vi "IR Opo Main.vi"() -> ()   [LabVIEW 2016]
uses:
  System.Windows.Forms
  D:/Fabrizio/Labview Projects/IR OPO Controller/Branches/XPS version/uc480DotNet.dll
  uc480DotNet.dll
  <vilib>/Utility/miscctls.llb/LVBoundsTypeDef.ctl
  <vilib>/Utility/config.llb/Write Key (Double).vi
  <vilib>/Utility/config.llb/Write Key (I32).vi
  <vilib>/Utility/config.llb/Read Key (String).vi
  <vilib>/Utility/config.llb/Read Key (Double).vi
  <vilib>/Utility/config.llb/Read Key (I32).vi
  <vilib>/vision/NI_Vision_Development_Module.lvlib
  <vilib>/Utility/config.llb/NI_LVConfig.lvlib
  OPOTEK.dll
panel:
  in  "Acceleration \n(mm/s²)":dbl=20.0
  out "Camera Status":string="Load parameter"
  in  "Save configuration":bool
  in  "Stages status":bool
  in  "Transparency":u8 max=80 step=1
  in  "Overlay MSI Image":bool
  in  "Home Axes":bool
  in  "Tune":bool
  out "Axis 2 Offset":dbl
  out "Axis 1 Offset":dbl
  out "Acceleration":dbl
  out "Velocity":dbl
  in  "Axis Initial Parameters":T1={"Velocity (units/seconds)"=1.0, "Acceleration (units/seconds²)"=20.0, "Minimum Jerk Time (seconds)"=0.005, "Maximum Jerk Time (seconds)"=0.009} {"Maximum Jerk Time (seconds)" format="%.6e"; "Minimum Jerk Time (seconds)" format="%.6e"; "Acceleration (units/seconds²)" format="%.6e"; "Velocity (units/seconds)" format="%.6e"}
  out "Axis 2":string
  out "Axis 1":string
  out "XPS_Address":string
  in  "Axes Manual Control":bool
  out "ROI Area \n(mm2)":dbl=4.035870075999999
  out "Default Wavelenght":i32
  out "Laser on/off array":bool[][](array[boolean])
  out "Commands array":string[][](array[string])
  in  "Exit Camera":bool
  in  "Width (µm)":i32=240
  in  "Y offset":i32=406 step=1
  in  "X offset":i32=693 step=1
  out "Processi time (sec)":i32=117
  in  "Processing time unit":string(combo)="sec"
  out "Process time":dbl=117.0
  in  "Mode":i32(ring) items=["RGB 32"=0, "RGB 24"=1, "Y8 Monochrom"=6]
  in  "Camera":refnum<k24>(container)
  in  "Init Camera":bool
  in  "Start Live":bool
  in  "Stop Live":bool
  in  "Load Parameter":bool
  out "Error Out":errorcluster caption="error"
  out "Bits/Pixel":i32=32
  out "Width":i32=1280
  out "Height":i32=1024
  out "Serial Number":string="4102944807"
  in  "Camera ID":i32
  in  "Zoom":dbl(ring)=1.5 items=["4X"=4.0, "2X"=2.0, "1.5X"=1.5, "1.25X"=1.25, "1X"=1.0]
  in  "Gain Boost":bool=TRUE
  in  "Snapshot":bool
  out "Output":picture
  in  "Exposure":dbl(slide)=99.80425000000001 min=0.049933333333333337 max=99.9166 step=0.049933333333333337 scale=0.049933333333333337..99.9166 scale format="%#.3g"
  in  "Framerate":dbl(slide)=10.002522802986672 min=0.5926462556135453 max=18.75159388548027 step=0.01754124778810128 scale=0.5926462556135453..18.75159388548027 scale format="%#.3g"
  in  "Pixelclock":i32(slide)=24 min=5 max=40 step=1 scale=5.0..40.0
  in  "error in (no error)":errorcluster
  out "error out":errorcluster
  in  "Precision (%)":dbl=1.0 min=1.0 max=100.0 step=1.0 format="%#_3g"
  out "Time array":dbl[][](array[numeric])
  in  "Process Image":bool
  in  "Pixel size":dbl=12.19 step=0.01
  in  "Speed (µm/s)":i32=1000
  in  "Heigth (µm)":i32=240
  in  "Height  step \ndivider":i32=2
  out "ROI container\nheigth (µm)":i32=2267
  out "ROI container\nwidth (µm)":i32=2267
  out "Source":T2(plugin-control)
  in  "Open \nManual":bool
  in  "Capture":bool
  out "Log":string
  out "Laser Operation":bool
  in  "Alignment \ndiode":bool
  in  "LASER":bool
  in  "LAMP":bool
  in  "Wavelength":dbl=2940.0 min=2600.0 max=3200.0 step=1.0
  out "error_Code 3":i32
  in  "Repetition \nRate":enum16{"1", "2", "5", "10", "20"}(ring)=enum."20"
  in  "Flash lamp - Q Switch delay (%)":i16(slide) min=0 max=100 scale=0.0..100.0 scale format="%#.1f"
  out "error_Code 2":i32
  out "Max":dbl=3200.0
  out "Min":dbl=2600.0
  out "error_Code":i32
  out "laserCOMPort":i32
  out "motorCOMPort":i32
  in  "EXIT":bool
  # "Laser Control"
  # "Stages Control"
  # "Camera Control"
  # "ROI Processing"
  # "Laser spot size and position"
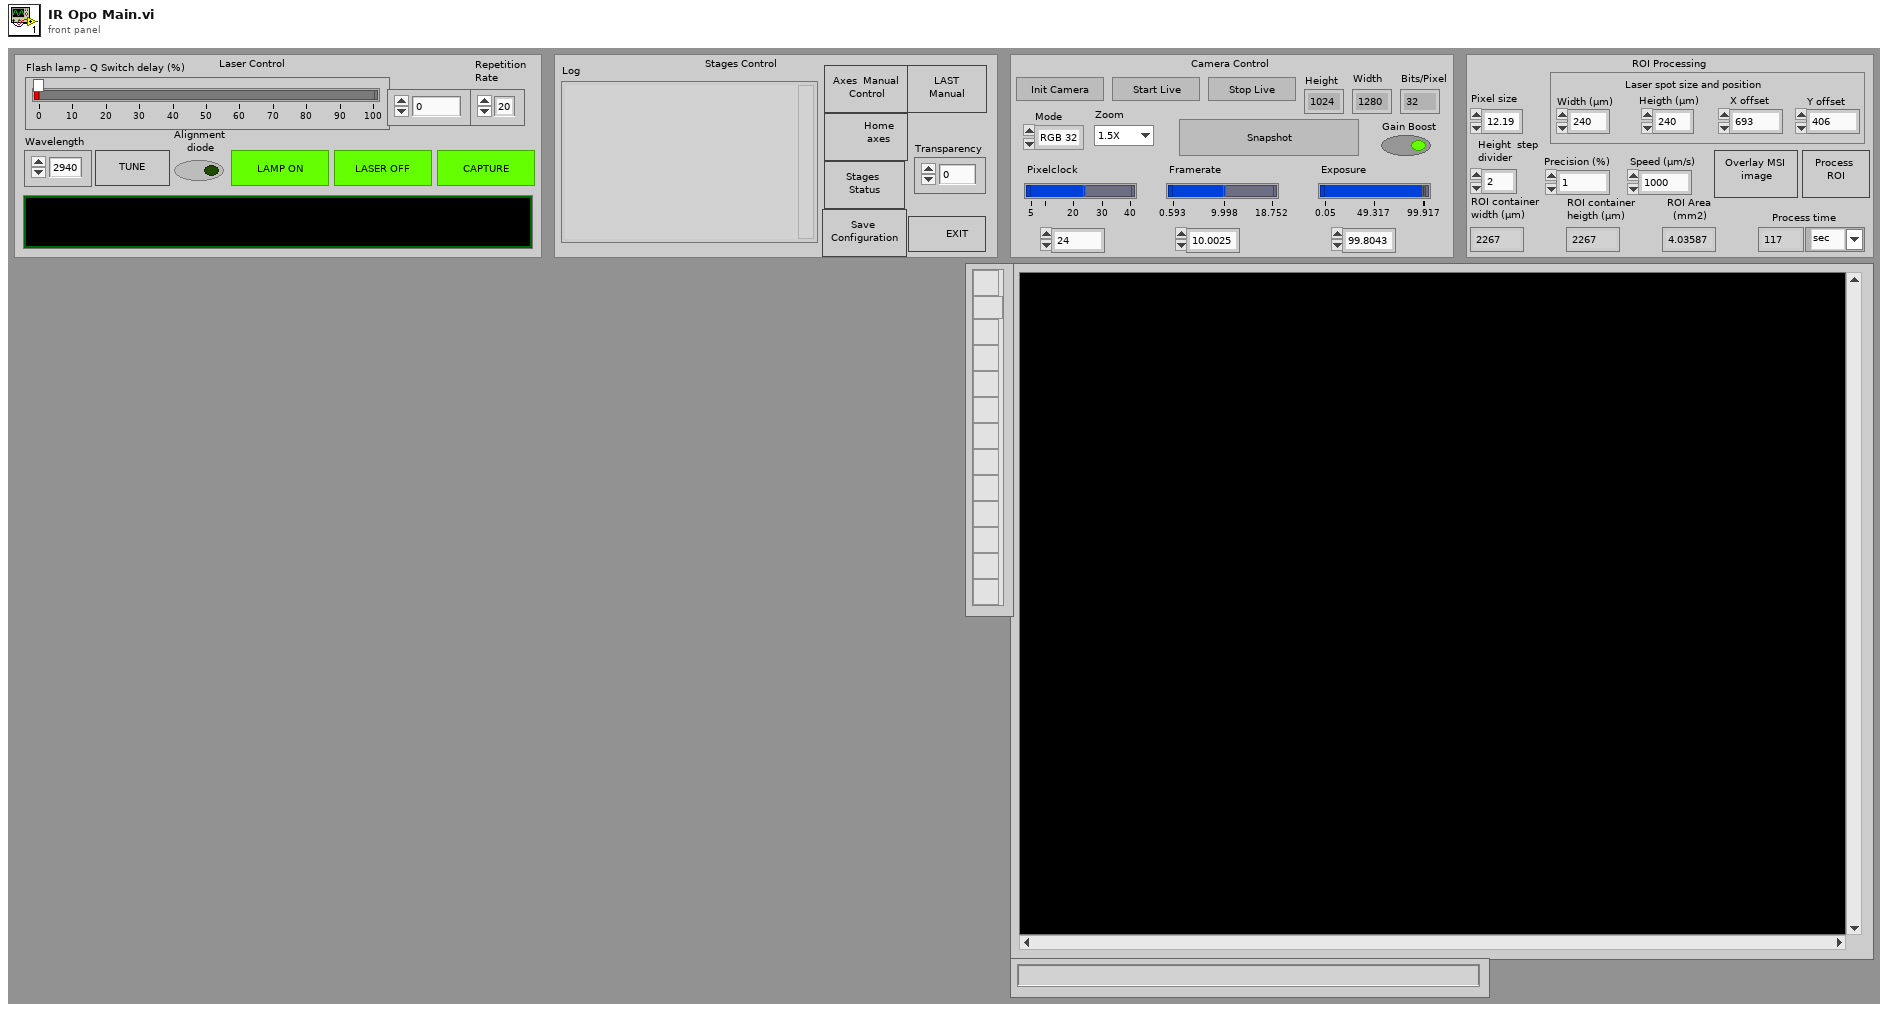
[diagram p1: front panel]
types:
  T1 = cluster{"Velocity (units/seconds)":dbl, "Acceleration (units/seconds²)":dbl, "Minimum Jerk Time (seconds)":dbl, "Maximum Jerk Time (seconds)":dbl}
  T2 = typedef "IMAQ Image.ctl" = refnum<image>
  T3 = typedef "LVBoundsTypeDef.ctl" = cluster{"Width":u32, "Height":u32}
  T4 = enum8{"Enabled", "Disabled", "Disabled and Grayed Out"}
  T5 = enum16{"Initialize", "Lamp ON", "Lamp OFF", "Q-switch ON", "Q-switch OFF", "Adjust Energy", "Change Rep. Rate", "Send String"}
  T6 = typedef "NI_LVConfig.lvlib/Config Data RefNum.ctl" = refnum<k1>
  T7 = cluster{"connection TCP":refnum<k5>, "LogTo File":bool, "Log File refnum":refnum<file>, "no error if error log":bool}
  T8 = enum16{"open", "replace", "create", "open or create", "replace or create", "replace or create with confirmation"}
  T9 = enum32{"Invalid", "Standard", "Closed", "Hidden", "Minimized", "Maximized"}
  T10 = enum32{"invalid app kind", "Development System", "Run Time System", "Student Edition", "Embedded LabVIEW", "Evaluation", "Custom"}
  T11 = typedef "Image Type" = u32
  T12 = cluster{"Global Rectangle":i32[], "Contours":cluster{"Contour Type":u32, "ROI Type":u32, "Points":i32[]}[]}
  T13 = cluster{"Global Rectangle[0]":i32, "Global Rectangle[1]":i32}
diagram:
  w36 = 1 items=["None", "FixedSingle", "Fixed3D"] ("BorderStyle")
  # "Button and controls"
  # "Camera control buttons"
  n1 = property class="PictureBox"(reference="Camera", "BorderStyle"=w36, "Width"=853, "Height"=682) -> (reference out=w24:refnum<k24>, error out=w25:errorcluster)  [unwired: 1 in]
  n2 = property class="PictureBox"(reference=w24, error in=w25) -> (reference out=w23:refnum<k24>, error out=w22:errorcluster, "Handle"=w21:refnum<k24>)
  n3 = while "Camera Control" {
    shift-right: [w53] -> _
    shift-left: w22 -> [w59]
    shift-right: [w56] -> _
    shift-left: _ -> [w49]
    shift-right: [w51] -> _
    shift-left: w23 -> [w52]
    tunnel: w21 -> [w50]
    stop <- w57 stop-if-true
    # ".NetReference"
    # ".Net Reference"
    n4 = event shown="[1] Timeout" {
      selector: _ -> [_ _]
      dyn-events: _ -> [_ _]
      timeout: 0 -> [_ _]
      event "Load Parameter", "Start Live": Mouse Down {
        n5 = event-data() -> ()  [unwired: 1 in, 2 out]
      }
      event Timeout {
        n6 = event-data() -> ()  [unwired: 1 in, 2 out]
      }
    }
    n7 = event shown="[1] Timeout" {
      selector: _ -> [_ _]
      dyn-events: _ -> [_ _]
      timeout: 0 -> [_ _]
      tunnel: [w73 w84] -> w60
      tunnel: w59 -> [w83 w84]
      tunnel: w49 -> [w82 _]
      event "Pixelclock": Value Change; "Pixelclock": Mouse Move; "Pixelclock": Key Down; "Pixelclock": Mouse Up {
        n8 = event-data() -> ("CtlRef"=w75:refnum<vi>)  [unwired: 1 in, 3 out]
        n9 = call "uc480_SubVI_Example_GetFramerate.vi"(".NET (Reference)"=w82, "Error In"=w83) -> ("Framerate"=w81:dbl, "Inc"=w80:dbl, "Min"=w78:dbl, "Max"=w79:dbl, "error out"=w77:errorcluster)  [unwired: 9 in]
        n10 = property on="Framerate" class="Slide (strict)"(error in=w77, "Value"=w81, "Increment"=w80, "Minimum"=w78, "Maximum"=w79) -> (error out=w76:errorcluster)  [unwired: 1 in, 1 out]
        n11 = property on="Framerate" class="Slide (strict)"(error in=w76, "Scale.Increment"=w80, "Scale.Minimum"=w78, "Scale.Maximum"=w79) -> (error out=w74:errorcluster)  [unwired: 1 in, 1 out]
        n12 = Close Reference(reference=w75, error in (no error)=w74) -> (error out=w73:errorcluster)
      }
      event Timeout {
        n13 = event-data() -> ()  [unwired: 1 in, 2 out]
      }
    }
    n14 = case shown="False" "Load Parameter" {
      tunnel: ["" "Load parameter"] -> w66
      frame False {
      }
      frame True {
      }
    }
    n15 = case shown="False" "Init Camera" {
      tunnel: ["" "Init camera"] -> w70
      frame False {
      }
      frame True {
      }
    }
    n16 = case shown="False" "Exit Camera" {
      tunnel: ["" "Exit camera"] -> w64
      frame False {
      }
      frame True {
      }
    }
    n17 = event shown="[1] Timeout" {
      selector: _ -> [_ _]
      dyn-events: _ -> [_ _]
      timeout: 0 -> [_ _]
      tunnel: w60 -> [w95 w96]
      tunnel: [w85 w96] -> w62
      tunnel: w49 -> [w94 _]
      event "Pixelclock", "Framerate": Value Change; "Pixelclock", "Framerate": Mouse Move; "Pixelclock", "Framerate": Key Down; "Pixelclock", "Framerate": Mouse Up {
        n18 = event-data() -> ("CtlRef"=w87:refnum<vi>)  [unwired: 1 in, 3 out]
        n19 = call "uc480_SubVI_Example_GetExposure.vi"(".NET (Reference)"=w94, "Error In"=w95) -> ("Exposure"=w91:dbl, "Inc"=w90:dbl, "Min"=w89:dbl, "Max"=w88:dbl, "Error out"=w92:errorcluster)  [unwired: 9 in]
        n20 = property on="Exposure" class="Slide (strict)"(error in=w92, "Value"=w91, "Increment"=w90, "Minimum"=w89, "Maximum"=w88) -> (error out=w93:errorcluster)  [unwired: 1 in, 1 out]
        n21 = property on="Exposure" class="Slide (strict)"(error in=w93, "Scale.Increment"=w90, "Scale.Minimum"=w89, "Scale.Maximum"=w88) -> (error out=w86:errorcluster)  [unwired: 1 in, 1 out]
        n22 = Close Reference(reference=w87, error in (no error)=w86) -> (error out=w85:errorcluster)
      }
      event Timeout {
        n23 = event-data() -> ()  [unwired: 1 in, 2 out]
      }
    }
    n24 = case shown="False" "Start Live" {
      tunnel: ["" "Start live"] -> w69
      frame False {
      }
      frame True {
      }
    }
    n25 = case shown="False" "Stop Live" {
      tunnel: ["" "Stop live"] -> w65
      frame False {
      }
      frame True {
      }
    }
    n26 = local read "Camera Status"() -> (w46:string)
    n27 = Concatenate Strings(w70, w69, w66, w65, w64) -> (→"Camera Status":string)
    n28 = case shown="Default" w46 {
      tunnel: w49 -> [w139 w179 w237 w279 w459 w518]
      tunnel: w62 -> [w142 w180 w238 w289 w458 w519]
      tunnel: [w113 w178 w246 w288 w417 w517] -> w56
      tunnel: [w114 w177 w247 w287 w454 w515] -> w55
      tunnel: [FALSE FALSE TRUE FALSE FALSE FALSE] -> w57
      tunnel: w52 -> [w112 w171 w219 w271 w412 w508]
      tunnel: [w112 w171 w218 w270 w412 w508] -> w51
      tunnel: w50 -> [_ _ _ w267 _ _]
      frame "Load parameter" {
        # "SubVI Example for \nMemory allocation"
        # "Is acquisition running?"
        # "Load Parameter"
        n29 = property class="Camera"(reference=w139, error in=w142) -> (error out=w147:errorcluster, "Acquisition"=w146:refnum<k24>)  [unwired: 1 out]
        n30 = invoke class="Acquisition" method="HasStarted"(reference=w146, error in=w147) -> (reference out=w143:refnum<k24>, error out=w145:errorcluster, "bValue"=w141:bool)  [unwired: 2 in, 1 out]
        n31 = control-ref of="Start Live"() -> (w137:refnum<vi>)
        n32 = invoke class="Acquisition" method="ToString"(reference=w143, error in=w145) -> (reference out=w109:refnum<k24>, error out=w108:errorcluster, "ToString"=w144:string)  [unwired: 1 in]
        n33 = property class="Bool"(reference=w137, "Disabled"=u8 0 ("Deaktiviert")) -> (reference out=w111:refnum<vi>, error out=w110:errorcluster)  [unwired: 1 in]
        n34 = Close Reference(reference=w109, error in (no error)=w108) -> (error out=w107:errorcluster)
        n35 = Close Reference(reference=w111, error in (no error)=w110) -> ()  [unwired: 1 out]
        n36 = call "uc480_Error_Handling.vi"("Error String"=w144, "Error In"=w107) -> ("Error Out"=w140:errorcluster)  [unwired: 9 in]
        n37 = case shown="False" w141 {
          tunnel: w140 -> [w155 w162]
          tunnel: w139 -> [w153 w163]
          tunnel: [w154 w162] -> w138
          tunnel: [w153 w163] -> w113
          frame False {
            n38 = property class="Camera"(reference=w153, error in=w155) -> (error out=w157:errorcluster, "Parameter"=w156:refnum<k24>)  [unwired: 1 out]
            n39 = invoke class="Parameter" method="Load"(reference=w156, error in=w157, "strFilename"="") -> (reference out=w159:refnum<k24>, error out=w160:errorcluster, "Load"=w152:i32)  [unwired: 1 in, 1 out]
            n40 = invoke class="Parameter" method="ToString"(reference=w159, error in=w160) -> (reference out=w149:refnum<k24>, error out=w151:errorcluster, "ToString"=w161:string)  [unwired: 1 in]
            n41 = Close Reference(reference=w149, error in (no error)=w151) -> (error out=w150:errorcluster)
            n42 = call "uc480_Error_Handling.vi"("Error Code"=w152, "Error String"=w161, "Error In"=w150) -> ("Error Out"=w154:errorcluster)  [unwired: 8 in]
          }
          frame True {
          }
        }
        n43 = call "uc480_SubVI_Example_MemoryAllocation.vi"(".NET (Reference)"=w113, "Error In"=w138) -> ("Error Out"=w115:errorcluster)  [unwired: 13 in, 4 out]
        n44 = call "uc480_SubVI_Example_GetPixelClock.vi"(".NET (Reference)"=w113, "Error In"=w115) -> ("Pixel Clock"=w116:i32, "Inc"=w118:i32, "Min"=w119:i32, "Max"=w120:i32, "error out"=w117:errorcluster)  [unwired: 9 in]
        n45 = property on="Pixelclock" class="Slide (strict)"(error in=w117, "Value"=w116, "Increment"=w118, "Minimum"=w119, "Maximum"=w120) -> (error out=w121:errorcluster)  [unwired: 1 in, 1 out]
        n46 = property on="Pixelclock" class="Slide (strict)"(error in=w121, "Scale.Increment"=w118, "Scale.Minimum"=w119, "Scale.Maximum"=w120) -> (error out=w122:errorcluster)  [unwired: 1 in, 1 out]
        n47 = call "uc480_SubVI_Example_GetFramerate.vi"(".NET (Reference)"=w113, "Error In"=w122) -> ("Framerate"=w125:dbl, "Inc"=w126:dbl, "Min"=w127:dbl, "Max"=w128:dbl, "error out"=w124:errorcluster)  [unwired: 9 in]
        n48 = property on="Framerate" class="Slide (strict)"(error in=w124, "Value"=w125, "Increment"=w126, "Minimum"=w127, "Maximum"=w128) -> (error out=w123:errorcluster)  [unwired: 1 in, 1 out]
        n49 = property on="Framerate" class="Slide (strict)"(error in=w123, "Scale.Increment"=w126, "Scale.Minimum"=w127, "Scale.Maximum"=w128) -> (error out=w129:errorcluster)  [unwired: 1 in, 1 out]
        n50 = call "uc480_SubVI_Example_GetExposure.vi"(".NET (Reference)"=w113, "Error In"=w129) -> ("Exposure"=w132:dbl, "Inc"=w133:dbl, "Min"=w134:dbl, "Max"=w135:dbl, "Error out"=w130:errorcluster)  [unwired: 9 in]
        n51 = property on="Exposure" class="Slide (strict)"(error in=w130, "Value"=w132, "Increment"=w133, "Minimum"=w134, "Maximum"=w135) -> (error out=w131:errorcluster)  [unwired: 1 in, 1 out]
        n52 = property on="Exposure" class="Slide (strict)"(error in=w131, "Scale.Increment"=w133, "Scale.Minimum"=w134, "Scale.Maximum"=w135) -> (error out=w114:errorcluster)  [unwired: 1 in, 1 out]
      }
      frame "Stop live" {
        # "Is acquisition running?"
        # "Stop Acquisition"
        n53 = property class="Camera"(reference=w179, error in=w180) -> (error out=w187:errorcluster, "Acquisition"=w186:refnum<k24>)  [unwired: 1 out]
        n54 = invoke class="Acquisition" method="HasStarted"(reference=w186, error in=w187) -> (reference out=w181:refnum<k24>, error out=w183:errorcluster, "bValue"=w185:bool)  [unwired: 2 in, 1 out]
        n55 = control-ref of="Load Parameter"() -> (w175:refnum<vi>)
        n56 = control-ref of="Start Live"() -> (w172:refnum<vi>)
        n57 = invoke class="Acquisition" method="ToString"(reference=w181, error in=w183) -> (reference out=w164:refnum<k24>, error out=w166:errorcluster, "ToString"=w182:string)  [unwired: 1 in]
        n58 = property class="Bool"(reference=w175, "Disabled"=u8 0 ("Deaktiviert")) -> (reference out=w170:refnum<vi>, error out=w169:errorcluster)  [unwired: 1 in]
        n59 = property class="Bool"(reference=w172, "Disabled"=u8 0 ("Deaktiviert")) -> (reference out=w168:refnum<vi>, error out=w167:errorcluster)  [unwired: 1 in]
        n60 = Close Reference(reference=w164, error in (no error)=w166) -> (error out=w165:errorcluster)
        n61 = Close Reference(reference=w170, error in (no error)=w169) -> ()  [unwired: 1 out]
        n62 = Close Reference(reference=w168, error in (no error)=w167) -> ()  [unwired: 1 out]
        n63 = call "uc480_Error_Handling.vi"("Error String"=w182, "Error In"=w165) -> ("Error Out"=w184:errorcluster)  [unwired: 9 in]
        n64 = case shown="True" w185 {
          tunnel: [w189 w208] -> w177
          tunnel: w184 -> [w189 w209]
          tunnel: w179 -> [w188 w201]
          tunnel: [w188 w201] -> w178
          frame False {
          }
          frame True {
            n65 = property class="Camera"(reference=w201, error in=w209) -> (error out=w205:errorcluster, "Acquisition"=w206:refnum<k24>)  [unwired: 1 out]
            n66 = invoke class="Acquisition" method="Stop"(reference=w206, error in=w205) -> (reference out=w203:refnum<k24>, error out=w204:errorcluster, "Stop"=w202:i32)  [unwired: 1 in]
            n67 = invoke class="Acquisition" method="ToString"(reference=w203, error in=w204) -> (reference out=w198:refnum<k24>, error out=w200:errorcluster, "ToString"=w207:string)  [unwired: 1 in]
            n68 = Close Reference(reference=w198, error in (no error)=w200) -> (error out=w199:errorcluster)
            n69 = call "uc480_Error_Handling.vi"("Error Code"=w202, "Error String"=w207, "Error In"=w199) -> ("Error Out"=w208:errorcluster)  [unwired: 8 in]
            n70 = Get Date/Time In Seconds() -> (seconds since 1Jan1904=w196:timestamp)
            n71 = Format Date/Time String(time format string (%c)="%m/%d/%y - %I:%M %p  ", seconds (now)=w196) -> (date/time string=w197:string)  [unwired: 1 in]
            n72 = Concatenate Strings(w197, "Camera stopped", "\r") -> (w192:string)
            n73 = invoke on="Log" class="Str" method="Append String"("string"=w192) -> (error out=w190:errorcluster)  [unwired: 3 in, 3 out]
            n74 = property on="Log" class="Str"(error in=w190, "Text.Scroll Position"=u32 500000) -> ()  [unwired: 1 in, 2 out]
          }
        }
      }
      frame "Exit camera" {
        # "Close .Net Reference"
        # "Is acquisition running?"
        # "Stop Acquisition"
        # "Close Camera"
        n75 = property class="Camera"(reference=w237, error in=w238) -> (error out=w245:errorcluster, "Acquisition"=w244:refnum<k24>)  [unwired: 1 out]
        n76 = invoke class="Acquisition" method="HasStarted"(reference=w244, error in=w245) -> (reference out=w239:refnum<k24>, error out=w241:errorcluster, "bValue"=w243:bool)  [unwired: 2 in, 1 out]
        n77 = control-ref of="Load Parameter"() -> (w228:refnum<vi>)
        n78 = control-ref of="Init Camera"() -> (w230:refnum<vi>)
        n79 = control-ref of="Start Live"() -> (w229:refnum<vi>)
        n80 = control-ref of="Stop Live"() -> (w227:refnum<vi>)
        n81 = invoke class="Acquisition" method="ToString"(reference=w239, error in=w241) -> (reference out=w224:refnum<k24>, error out=w226:errorcluster, "ToString"=w240:string)  [unwired: 1 in]
        n82 = property class="Bool"(reference=w229, "Disabled"=u8 0 ("Deaktiviert")) -> (reference out=w213:refnum<vi>, error out=w212:errorcluster)  [unwired: 1 in]
        n83 = property class="Bool"(reference=w230, "Disabled"=u8 0 ("Deaktiviert")) -> (reference out=w211:refnum<vi>, error out=w210:errorcluster)  [unwired: 1 in]
        n84 = property class="Bool"(reference=w228, "Disabled"=u8 0 ("Deaktiviert")) -> (reference out=w215:refnum<vi>, error out=w214:errorcluster)  [unwired: 1 in]
        n85 = property class="Bool"(reference=w227, "Disabled"=u8 0 ("Deaktiviert")) -> (reference out=w217:refnum<vi>, error out=w216:errorcluster)  [unwired: 1 in]
        n86 = Close Reference ("Close Referenz")(reference=w224, error in (no error)=w226) -> (error out=w225:errorcluster)
        n87 = Close Reference(reference=w213, error in (no error)=w212) -> ()  [unwired: 1 out]
        n88 = Close Reference(reference=w211, error in (no error)=w210) -> ()  [unwired: 1 out]
        n89 = Close Reference(reference=w217, error in (no error)=w216) -> ()  [unwired: 1 out]
        n90 = Close Reference(reference=w215, error in (no error)=w214) -> ()  [unwired: 1 out]
        n91 = call "uc480_Error_Handling.vi"("Error String"=w240, "Error In"=w225) -> ("Error Out"=w242:errorcluster)  [unwired: 9 in]
        n92 = case shown="True" w243 {
          tunnel: [w254 w265] -> w235
          tunnel: w242 -> [w254 w266]
          tunnel: w237 -> [w253 w258]
          tunnel: [w253 w258] -> w236
          frame False {
          }
          frame True {
            n93 = property class="Camera"(reference=w258, error in=w266) -> (error out=w262:errorcluster, "Acquisition"=w263:refnum<k24>)  [unwired: 1 out]
            n94 = invoke class="Acquisition" method="Stop"(reference=w263, error in=w262) -> (reference out=w260:refnum<k24>, error out=w261:errorcluster, "Stop"=w259:i32)  [unwired: 1 in]
            n95 = invoke class="Acquisition" method="ToString"(reference=w260, error in=w261) -> (reference out=w255:refnum<k24>, error out=w257:errorcluster, "ToString"=w264:string)  [unwired: 1 in]
            n96 = Close Reference ("Close Referenz")(reference=w255, error in (no error)=w257) -> (error out=w256:errorcluster)
            n97 = call "uc480_Error_Handling.vi"("Error Code"=w259, "Error String"=w264, "Error In"=w256) -> ("Error Out"=w265:errorcluster)  [unwired: 8 in]
          }
        }
        n98 = invoke class="Camera" method="Exit"(reference=w236, error in=w235) -> (reference out=w246:refnum<k24>, error out=w249:errorcluster, "Exit"=w248:i32)  [unwired: 1 in]
        n99 = invoke class="Camera" method="ToString"(reference=w246, error in=w249) -> (error out=w250:errorcluster, "ToString"=w251:string)  [unwired: 1 in, 1 out]
        n100 = call "uc480_Error_Handling.vi"("Error Code"=w248, "Error String"=w251, "Error In"=w250) -> ("Error Out"=w223:errorcluster)  [unwired: 8 in]
        n101 = property class="PictureBox"(reference=w219, error in=w223, "Width"=853, "Height"=682) -> (reference out=w218:refnum<k24>, error out=w222:errorcluster)
        n102 = Close Reference ("Close Referenz")(reference=w246, error in (no error)=w222) -> (error out=w247:errorcluster)
      }
      frame Default {
        # "SubVI Example for Timing"
        # "Has acquisition started?"
        n103 = call "uc480_SubVI_Example_Timing.vi"(".NET (Reference)"=w279, "Pixelclock"="Pixelclock", "Exposure time"="Exposure", "Framerate"="Framerate", "Error In"=w289) -> ("Pixelclock"=w282:i32, "Exposure time"=w281:dbl, "Framerate"=w280:dbl, "Error Out"=w286:errorcluster)  [unwired: 7 in]
        n104 = property on="Framerate" class="Schieber (strikt)"(error in=w286, "Scale.RngStart"=w280) -> (error out=w285:errorcluster)  [unwired: 1 in, 1 out]
        n105 = property on="Exposure" class="Schieber (strikt)"(error in=w285, "Scale.RngStart"=w281) -> (error out=w284:errorcluster)  [unwired: 1 in, 1 out]
        n106 = property on="Pixelclock" class="Schieber (strikt)"(error in=w284, "Scale.RngStart"=w282) -> (error out=w283:errorcluster)  [unwired: 1 in, 1 out]
        n107 = property class="Camera"(reference=w279, error in=w283) -> (reference out=w272:refnum<k24>, error out=w295:errorcluster, "Acquisition"=w294:refnum<k24>)
        n108 = invoke class="Acquisition" method="HasStarted"(reference=w294, error in=w295) -> (reference out=w269:refnum<k24>, error out=w291:errorcluster, "HasStarted"=w290:i32, "bValue"=w268:bool)  [unwired: 2 in]
        n109 = invoke class="Acquisition" method="ToString"(reference=w269, error in=w291) -> (reference out=w273:refnum<k24>, error out=w293:errorcluster, "ToString"=w292:string)  [unwired: 1 in]
        n110 = call "uc480_Error_Handling.vi"("Error Code"=w290, "Error String"=w292, "Error In"=w293) -> ("Error Out"=w275:errorcluster)  [unwired: 8 in]
        n111 = Close Reference(reference=w273, error in (no error)=w275) -> (error out=w274:errorcluster)
        n112 = case "Show Image" shown="False" w268 {
          tunnel: [w299 w311] -> w287
          tunnel: w274 -> [w299 w339]
          tunnel: w272 -> [w298 w303]
          tunnel: [w298 w307] -> w288
          tunnel: w271 -> [w297 w328]
          tunnel: [w297 w305] -> w270
          tunnel: w267 -> [_ w335]
          frame False {
            (unwired) ""
          }
          frame True {
            n113 = local read "Height"() -> (w332:i32)
            n114 = local read "Width"() -> (w333:i32)
            n115 = Quotient & Remainder(x=w333, y="Zoom") -> (floor(x/y)=w330:dbl)  [unwired: 1 out]
            n116 = Quotient & Remainder(x=w332, y="Zoom") -> (floor(x/y)=w329:dbl)  [unwired: 1 out]
            n117 = To Long Integer(number=w330) -> (32bit integer=w302:i32)
            n118 = To Long Integer(number=w329) -> (32bit integer=w301:i32)
            n119 = property class="PictureBox"(reference=w328, error in=w339, "Width"=w302, "Height"=w301) -> (reference out=w305:refnum<k24>, error out=w334:errorcluster)
            n120 = property class="Camera"(reference=w303, error in=w334) -> (reference out=w304:refnum<k24>, error out=w341:errorcluster, "Memory"=w342:refnum<k24>)
            n121 = invoke class="Memory" method="GetActive"(reference=w342, error in=w341) -> (reference out=w336:refnum<k24>, error out=w337:errorcluster, "s32MemId"=w308:i32)  [unwired: 2 in, 1 out]
            n122 = property class="Camera"(reference=w304, error in=w337) -> (reference out=w316:refnum<k24>, error out=w340:errorcluster, "Display"=w325:refnum<k24>)
            n123 = invoke class="Display" method="Render"(reference=w325, error in=w340, "memID"=w308, "windowHandle"=w335) -> (reference out=w326:refnum<k24>, error out=w327:errorcluster)  [unwired: 1 in, 3 out]
            n124 = property class="Camera"(reference=w316, error in=w327) -> (reference out=w307:refnum<k24>, error out=w323:errorcluster, "Gain"=w321:refnum<k24>)
            n125 = property class="Gain"(reference=w321, error in=w323) -> (reference out=w322:refnum<k24>, error out=w318:errorcluster, "Hardware"=w317:refnum<k24>)
            n126 = property class="GainHardware"(reference=w317, error in=w318) -> (reference out=w314:refnum<k24>, error out=w319:errorcluster, "Boost"=w320:refnum<k24>)
            n127 = property class="GainBoost"(reference=w320, error in=w319, "Enabled"="Gain Boost") -> (reference out=w315:refnum<k24>, error out=w306:errorcluster)
            n128 = case "Snapshot control" shown="False" "Snapshot" {
              tunnel: w303 -> [_ w363]
              tunnel: w306 -> [w343 w367]
              tunnel: [w343 w354] -> w300
              tunnel: w302 -> [_ w357]
              tunnel: w301 -> [_ w356]
              frame False {
              }
              frame True {
                n129 = property class="Camera"(reference=w363, error in=w367) -> (error out=w387:errorcluster, "Memory"=w386:refnum<k24>)  [unwired: 1 out]
                n130 = local read "Zoom"() -> (w362:dbl)
                n131 = invoke class="Memory" method="GetList"(reference=w386, error in=w387) -> (reference out=w392:refnum<k24>, error out=w391:errorcluster, "GetList"=w393:i32, "idList"=w380:i32[])  [unwired: 2 in]
                n132 = Bundle(cluster=T3 {"Width"=0, "Height"=0} ("Draw Area Size"), "Width"=w357, "Height"=w356) -> (w358:T3)
                n133 = Divide(x=1.0, y=w362) -> (x/y=w360:dbl)
                n134 = property on="Output" class="Pict"("ZoomFactor"=w360, "Draw Area Size"=w358) -> ()  [unwired: 2 in, 2 out]
                n135 = invoke class="Memory" method="ToString"(reference=w392, error in=w391) -> (reference out=w365:refnum<k24>, error out=w375:errorcluster, "ToString"=w390:string)  [unwired: 1 in]
                n136 = Index Array(array=w380, index=0 ("Active \nAcquisition Buffer")) -> (element=w377:i32)
                n137 = Index Array(array=w380, index=u32 0 ("Active \nOutput Buffer")) -> (element=w376:i32)
                n138 = Close Reference(reference=w365, error in (no error)=w375) -> (error out=w374:errorcluster)
                n139 = call "uc480_Error_Handling.vi"("Error Code"=w393, "Error String"=w390, "Error In"=w374) -> ("Error Out"=w383:errorcluster)  [unwired: 8 in]
                n140 = Get Date/Time In Seconds() -> (seconds since 1Jan1904=w347:timestamp)
                n141 = property class="Camera"(reference=w363, error in=w383) -> (error out=w382:errorcluster, "Memory"=w381:refnum<k24>)  [unwired: 1 out]
                n142 = Format Date/Time String(time format string (%c)="%m/%d/%y -%I:%M %p  ", seconds (now)=w347) -> (date/time string=w346:string)  [unwired: 1 in]
                n143 = invoke class="Memory" method="SetActive"(reference=w381, error in=w382, "s32MemId"=w377) -> (reference out=w366:refnum<k24>, error out=w373:errorcluster)  [unwired: 1 in, 2 out]
                n144 = Concatenate Strings(w346, "Snapshot taken", "\r") -> (w351:string)
                n145 = Close Reference(reference=w366, error in (no error)=w373) -> (error out=w372:errorcluster)
                n146 = invoke on="Log" class="Str" method="Append String"("string"=w351) -> (error out=w344:errorcluster)  [unwired: 3 in, 3 out]
                n147 = property class="Camera"(reference=w363, error in=w372) -> (error out=w389:errorcluster, "Memory"=w378:refnum<k24>)  [unwired: 1 out]
                n148 = invoke class="Memory" method="CopyToArray"(reference=w378, error in=w389, "s32MemId"=w376) -> (reference out=w368:refnum<k24>, error out=w369:errorcluster, "u8Image"=w388:u8[])  [unwired: 2 in, 2 out]
                n149 = property on="Log" class="Str"(error in=w344, "Text.Scroll Position"=u32 500000) -> ()  [unwired: 1 in, 2 out]
                n150 = invoke class="Memory" method="ToString"(reference=w368, error in=w369) -> (reference out=w364:refnum<k24>, error out=w371:errorcluster, "ToString"=w394:string)  [unwired: 1 in]
                n151 = Close Reference(reference=w364, error in (no error)=w371) -> (error out=w370:errorcluster)
                n152 = call "uc480_Error_Handling.vi"("Error String"=w394, "Error In"=w370) -> ("Error Out"=w385:errorcluster)  [unwired: 9 in]
                n153 = call "uc480_ArrayToImage.vi"("Error In"=w385, "InArray"=w388, ".NET (Reference)"=w363) -> ("Error Out"=w353:errorcluster, "Image"=w355:picture)  [unwired: 7 in]
                "Output" <- w355
                n154 = call "Picture to IMAQ.vi"("Error In"=w353, "picture"=w355) -> ("Error Out"=w354:errorcluster, "Image"=→"Source":T2)  [unwired: 8 in]
              }
            }
            n155 = Close Reference(reference=w314, error in (no error)=w300) -> (error out=w313:errorcluster)
            n156 = Close Reference(reference=w315, error in (no error)=w313) -> (error out=w310:errorcluster)
            n157 = Close Reference(reference=w322, error in (no error)=w310) -> (error out=w324:errorcluster)
            n158 = Close Reference(reference=w326, error in (no error)=w324) -> (error out=w338:errorcluster)
            n159 = Close Reference(reference=w336, error in (no error)=w338) -> (error out=w311:errorcluster)
          }
        }
      }
      frame "Init camera" {
        # "SubVI Example for \nGetDefault Timing"
        # "SubVI Example for \nMemory allocation"
        # "SubVI Example for \nTiming"
        # "SubVI Example for \nCamera Init"
        # "Pixelformat"
        n160 = control-ref of="Load Parameter"() -> (w418:refnum<vi>)
        n161 = call "uc480_SubVI_Example_CameraInit.vi"("Error In"=w458, "Camera ID"="Camera ID", "Init Camera Flag"=TRUE, ".NET (Reference)"=w459) -> ("Error Out"=w464:errorcluster, ".NET (Reference)"=w417:refnum<k24>)  [unwired: 6 in]
        n162 = control-ref of="Init Camera"() -> (w422:refnum<vi>)
        n163 = control-ref of="Start Live"() -> (w420:refnum<vi>)
        n164 = property on="Property Node" class="Camera"(reference=w417, error in=w464) -> (error out=w465:errorcluster, "PixelFormat"=w466:refnum<k24>)  [unwired: 1 out]
        n165 = property class="Bool"(reference=w420, "Disabled"=u8 0 ("Deaktiviert")) -> (reference out=w409:refnum<vi>, error out=w408:errorcluster)  [unwired: 1 in]
        n166 = property class="Bool"(reference=w422, "Disabled"=u8 2 ("Deaktiviert")) -> (reference out=w411:refnum<vi>, error out=w410:errorcluster)  [unwired: 1 in]
        n167 = property class="Bool"(reference=w418, "Disabled"=u8 0 ("Deaktiviert")) -> (reference out=w407:refnum<vi>, error out=w406:errorcluster)  [unwired: 1 in]
        n168 = Close Reference(reference=w409, error in (no error)=w408) -> ()  [unwired: 1 out]
        n169 = Close Reference(reference=w411, error in (no error)=w410) -> ()  [unwired: 1 out]
        n170 = Close Reference(reference=w407, error in (no error)=w406) -> ()  [unwired: 1 out]
        n171 = invoke class="PixelFormat" method="Set"(reference=w466, error in=w465, "mode"="Mode") -> (reference out=w462:refnum<k24>, error out=w455:errorcluster, "Set"=w461:i32)  [unwired: 1 in, 1 out]
        n172 = Get Date/Time In Seconds() -> (seconds since 1Jan1904=w398:timestamp)
        n173 = Format Date/Time String(time format string (%c)="%m/%d/%y - %I:%M %p  ", seconds (now)=w398) -> (date/time string=w397:string)  [unwired: 1 in]
        n174 = invoke class="PixelFormat" method="ToString"(reference=w462, error in=w455) -> (reference out=w403:refnum<k24>, error out=w405:errorcluster, "ToString"=w463:string)  [unwired: 1 in]
        n175 = Concatenate Strings(w397, "Camera Initialized", "\r") -> (w402:string)
        n176 = Close Reference(reference=w403, error in (no error)=w405) -> (error out=w404:errorcluster)
        n177 = call "uc480_Error_Handling.vi"("Error Code"=w461, "Error String"=w463, "Error In"=w404) -> ("Error Out"=w429:errorcluster)  [unwired: 8 in]
        n178 = invoke on="Log" class="Str" method="Append String"("string"=w402) -> (error out=w395:errorcluster)  [unwired: 3 in, 3 out]
        n179 = property on="Log" class="Str"(error in=w395, "Text.Scroll Position"=u32 500000) -> ()  [unwired: 1 in, 2 out]
        n180 = call "uc480_SubVI_Example_GetDefault_Timing.vi"(".NET (Reference)"=w417, "Error In"=w429) -> ("Pixelclock"=w428:i32, "Exposure time"=w427:dbl, "Framerate"=w426:dbl, "Error Out"=w425:errorcluster)  [unwired: 10 in]
        n181 = call "uc480_SubVI_Example_GetPixelClock.vi"(".NET (Reference)"=w417, "Error In"=w425) -> ("Pixel Clock"=w430:i32, "Inc"=w432:i32, "Min"=w433:i32, "Max"=w434:i32, "error out"=w431:errorcluster)  [unwired: 9 in]
        n182 = property on="Pixelclock" class="Slide (strict)"(error in=w431, "Value"=w430, "Increment"=w432, "Minimum"=w433, "Maximum"=w434) -> (error out=w435:errorcluster)  [unwired: 1 in, 1 out]
        n183 = property on="Pixelclock" class="Slide (strict)"(error in=w435, "Scale.Increment"=w432, "Scale.Minimum"=w433, "Scale.Maximum"=w434) -> (error out=w436:errorcluster)  [unwired: 1 in, 1 out]
        n184 = call "uc480_SubVI_Example_GetFramerate.vi"(".NET (Reference)"=w417, "Error In"=w436) -> ("Framerate"=w439:dbl, "Inc"=w440:dbl, "Min"=w441:dbl, "Max"=w442:dbl, "error out"=w438:errorcluster)  [unwired: 9 in]
        n185 = property on="Framerate" class="Slide (strict)"(error in=w438, "Value"=w439, "Increment"=w440, "Minimum"=w441, "Maximum"=w442) -> (error out=w437:errorcluster)  [unwired: 1 in, 1 out]
        n186 = property on="Framerate" class="Slide (strict)"(error in=w437, "Scale.Increment"=w440, "Scale.Minimum"=w441, "Scale.Maximum"=w442) -> (error out=w443:errorcluster)  [unwired: 1 in, 1 out]
        n187 = call "uc480_SubVI_Example_GetExposure.vi"(".NET (Reference)"=w417, "Error In"=w443) -> ("Exposure"=w446:dbl, "Inc"=w447:dbl, "Min"=w448:dbl, "Max"=w449:dbl, "Error out"=w444:errorcluster)  [unwired: 9 in]
        n188 = property on="Exposure" class="Slide (strict)"(error in=w444, "Value"=w446, "Increment"=w447, "Minimum"=w448, "Maximum"=w449) -> (error out=w445:errorcluster)  [unwired: 1 in, 1 out]
        n189 = property on="Exposure" class="Slide (strict)"(error in=w445, "Scale.Increment"=w447, "Scale.Minimum"=w448, "Scale.Maximum"=w449) -> (error out=w424:errorcluster)  [unwired: 1 in, 1 out]
        n190 = call "uc480_SubVI_Example_Timing.vi"(".NET (Reference)"=w417, "Pixelclock"=w428, "Exposure time"=w427, "Framerate"=w426, "Error In"=w424) -> ("Error Out"=w416:errorcluster)  [unwired: 7 in, 3 out]
        n191 = call "uc480_SubVI_Example_Is_XS.vi"("Error In"=w416, ".NET (Reference)"=w417) -> ("Error Out"=w413:errorcluster, "IsXS"=w415:bool)  [unwired: 7 in, 1 out]
        n192 = case shown="False" w415 {
          tunnel: w413 -> [w480 w493]
          tunnel: [w480 w493] -> w414
          frame False {
            n193 = control-ref of="Pixelclock"() -> (w476:refnum<vi>)
            n194 = control-ref of="Framerate"() -> (w475:refnum<vi>)
            n195 = control-ref of="Exposure"() -> (w474:refnum<vi>)
            n196 = property class="Slide (strict)"(reference=w476, "DisabledEnum"=T4."Enabled" ("Disabled")) -> (reference out=w473:refnum<vi>, error out=w472:errorcluster)  [unwired: 1 in]
            n197 = property class="Slide (strict)"(reference=w475, "DisabledEnum"=T4."Enabled" ("Disabled")) -> (reference out=w471:refnum<vi>, error out=w470:errorcluster)  [unwired: 1 in]
            n198 = property class="Slide (strict)"(reference=w474, "DisabledEnum"=T4."Enabled" ("Disabled")) -> (reference out=w469:refnum<vi>, error out=w468:errorcluster)  [unwired: 1 in]
            n199 = Close Reference(reference=w473, error in (no error)=w472) -> ()  [unwired: 1 out]
            n200 = Close Reference(reference=w471, error in (no error)=w470) -> ()  [unwired: 1 out]
            n201 = Close Reference(reference=w469, error in (no error)=w468) -> ()  [unwired: 1 out]
          }
          frame True {
            n202 = control-ref of="Pixelclock"() -> (w492:refnum<vi>)
            n203 = control-ref of="Framerate"() -> (w489:refnum<vi>)
            n204 = control-ref of="Exposure"() -> (w487:refnum<vi>)
            n205 = property class="Slide (strict)"(reference=w492, "DisabledEnum"=T4."Disabled and Grayed Out" ("Disabled")) -> (reference out=w485:refnum<vi>, error out=w486:errorcluster)  [unwired: 1 in]
            n206 = property class="Slide (strict)"(reference=w489, "DisabledEnum"=T4."Disabled and Grayed Out" ("Disabled")) -> (reference out=w484:refnum<vi>, error out=w483:errorcluster)  [unwired: 1 in]
            n207 = property class="Slide (strict)"(reference=w487, "DisabledEnum"=T4."Disabled and Grayed Out" ("Disabled")) -> (reference out=w482:refnum<vi>, error out=w481:errorcluster)  [unwired: 1 in]
            n208 = Close Reference(reference=w485, error in (no error)=w486) -> ()  [unwired: 1 out]
            n209 = Close Reference(reference=w484, error in (no error)=w483) -> ()  [unwired: 1 out]
            n210 = Close Reference(reference=w482, error in (no error)=w481) -> ()  [unwired: 1 out]